vi "UHR-Fleezers Control (host) - 10.8MV_trial1.vi"() -> ()   [LabVIEW 2010] (continued)
        n694 = xnode "Read/Write Control"("FPGA VI Reference In"=w3318, "error in"=w3316, "Green interlace ON count"="GI Frequency, ON count", "Green interlace OFF count"="GI Frequency, OFF count", "Green interlace ON count 2"="GI Frequency, ON count", "Green interlace OFF count 2"="GI Frequency, OFF count", "Green FB Count"="Green FB Count") -> ("error out"=w3317:errorcluster)  [unwired: 1 out]
      }
      event "Number of F/B Scans (AOD)", "Scan Speed (nm/s)", "Scan BD", "Initial delta (MHz)", "Step Size (nm)", "Scan Range (nm)": Value Change {
        w3497 = 123.0  # AOM cal (nm/MHz)
        n695 = event-data() -> ()  [unwired: 7 out]
        n696 = local read "BD 1 Frequency 1 (MHz)"() -> (w3480:dbl)
        n697 = local read "AOM X Cal (nm/MHz)"() -> (w3472:dbl)
        n698 = local read "X RF Frequency Limits (MHz)"() -> (w3484:T16)
        n699 = local read "Y RF Frequency Limits (MHz)"() -> (w3481:T16)
        n700 = local read "BD 2 Frequency 1 (MHz)"() -> (w3486:dbl)
        n701 = Negate(x="Scan Range (nm)") -> (-x=w3450:dbl)
        n702 = Divide(x=w3450, y=w3472) -> (x/y=w3454:dbl)
        n703 = Select(t=w3484, s="Scan BD", f=w3481) -> (s? t:f=w3483:T16)
        n704 = Select(t=w3480, s="Scan BD", f=w3486) -> (s? t:f=w3485:dbl)
        n705 = Unbundle By Name(w3483) -> ("Maximum"=w3492:dbl, "Minimum"=w3491:dbl)
        n706 = Add(x=w3454, y=w3485) -> (x+y=w3489:dbl)
        n707 = Divide(x=w3450, y="Step Size (nm)") -> (x/y=w3469:dbl)
        n708 = Divide(x="Step Size (nm)", y=w3472) -> (x/y=w3478:dbl)
        n709 = Absolute Value(x=w3469) -> (abs(x)=w3453:dbl)
        n710 = Sign(1:w3450) -> (0:w3451:dbl)
        n711 = In Range and Coerce(upper limit=w3492, x=w3489, lower limit=w3491) -> (coerced(x)=w3488:dbl, In Range?=w3490:bool)
        n712 = To Unsigned Quad Integer(1:w3453) -> (0:w3468:u64)
        "Scan steps (AOD)" <- w3468
        n713 = call "IR AOM freq to word.vi"("Frequency In (MHz)"=w3478) -> ("Frequency Word Out (double)"=w3475:dbl)
        n714 = Multiply(x=w3451, y=w3475) -> (x*y=w3452:dbl)
        n715 = Subtract(x=w3489, y=w3488) -> (x-y=w3487:dbl)
        n716 = To Quad Integer(1:w3452) -> (0:w3474:i64)
        "Incr. int (AOD)" <- w3474
        n717 = Subtract(x=w3454, y=w3487) -> (x-y=w3473:dbl)
        "Scan Range (MHz)" <- w3473
        n718 = Select(t=w3454, s=w3490, f=w3473) -> (s? t:f=w3493:dbl)
        n719 = Multiply(x=w3473, y=w3472) -> (x*y=w3471:dbl)
        n720 = Decrement(x=w3468) -> (x-1=w3521:u64)
        n721 = Negate(x=w3471) -> (-x=w3467:dbl)
        n722 = local write "Scan Range (nm)"(w3467) -> ()
        n723 = Divide(x=w3493, y=w3521) -> (x/y=w3477:dbl)
        "Scan Increment (MHz)" <- w3477
        n724 = call "IR AOM freq to word.vi"("Frequency In (MHz)"=w3477) -> ("Frequency Word Out (double)"=w3476:dbl)
        n725 = Divide(x="Step Size (nm)", y="Scan Speed (nm/s)") -> (x/y=w3464:dbl)
        n726 = To Quad Integer(1:w3476) -> ()  [unwired: 1 out]
        n727 = local read "Number Interlace Sets"() -> (w3448:u8)
        n728 = local read "AI Count (ticks)"() -> (w3449:u32)
        n729 = local read "Total Counts (ticks)"() -> (w3447:u32)
        n730 = local read "# Samples/trap"() -> (w3479:u32)
        n731 = Multiply(x=w3449, y=w3448) -> (x*y=w3446:u32)
        n732 = Divide(x=w3447, y=w3446) -> (x/y=w3445:dbl)
        n733 = Select(t=w3480, s="Scan BD", f=w3486) -> (s? t:f=w3518:dbl)
        "Initial freq. (MHz)" <- w3518
        n734 = Add(x=w3493, y=w3518) -> (x+y=→"Final freq. (MHz)":dbl)
        n735 = Divide(x=w3447, y=40000000.0) -> (x/y=w3463:dbl)
        n736 = Divide(x=w3464, y=w3463) -> (x/y=w3462:dbl)
        n737 = To Unsigned Quad Integer(1:w3462) -> (0:w3437:u64)
        n738 = Quotient & Remainder(x=w3437, y=u64 2) -> (x-y*floor(x/y)=w3441:u64)  [unwired: 1 out]
        n739 = Equal?(x=w3441, y=u64 0) -> (x = y?=w3439:bool)
        n740 = Decrement(x=w3437) -> (x-1=w3438:u64)
        n741 = Select(t=w3437, s=w3439, f=w3438) -> (s? t:f=w3436:u64)
        "Cycles/step (AOD)" <- w3436
        n742 = xnode "Read/Write Control"("FPGA VI Reference In"=w3529, "error in"=w3528, "Scan steps"=w3468, "Number of scans"="Number of F/B Scans (AOD)", "Cycles per step"=w3436, "Scan freq.  increment"=w3474, "Scan BD"="Scan BD") -> ("error out"=w3527:errorcluster)  [unwired: 1 out]
        n743 = Multiply(x=w3468, y=w3436) -> (x*y=w3522:u64)
        n744 = Multiply(x=w3522, y=u64 2) -> (x*y=w3444:u64)
        n745 = Multiply(x=w3445, y=w3444) -> (x*y=w3443:dbl)
        "Data points/scan (f/b)" <- w3443
        n746 = Multiply(x=w3443, y="Number of F/B Scans (AOD)") -> (x*y=w3525:dbl)
        "Data points/scans" <- w3525
        n747 = Divide(x=w3525, y=w3479) -> (x/y=→"N sets should be saved":dbl)
        n748 = Multiply(x=w3522, y=w3463) -> (x*y=w3461:dbl)
        "Time/Scan (s) (AOD)" <- w3461
        n749 = Select(t=w3493, s="Scan BD", f=0.0) -> (s? t:f=w3519:dbl)
        n750 = Select(t=0.0, s="Scan BD", f=w3493) -> (s? t:f=w3515:dbl)
        n751 = local read "BD 2 Frequency 2 (MHz)"() -> (w3511:dbl)
        n752 = local read "BD 1 Frequency 2 (MHz)"() -> (w3514:dbl)
        n753 = Add(x=w3515, y=w3486) -> (x+y=w3512:dbl)
        n754 = Add(x=w3480, y=w3519) -> (x+y=w3513:dbl)
        n755 = Multiply(x=w3461, y=2.0) -> (x*y=w3460:dbl)
        n756 = Multiply(x=w3460, y="Number of F/B Scans (AOD)") -> (x*y=w3457:dbl)
        n757 = Divide(x=w3457, y=60.0) -> (x/y=→"Time to Finish All (min)":dbl)
        n758 = Add(x="Trap 2 Bead Size (nm)", y="Trap 1 Bead Size (nm)") -> (x+y=w3501:dbl)
        n759 = local read "Initial delta (MHz)"() -> (w3498:dbl)
        n760 = Divide(x=w3501, y=2.0) -> (x/y=w3495:dbl)
        n761 = Subtract(x=w3512, y=w3511) -> (x-y=w3509:dbl)
        n762 = Subtract(x=w3513, y=w3514) -> (x-y=w3510:dbl)
        n763 = Square(x=w3509) -> (x^2=w3508:dbl)
        n764 = Square(x=w3510) -> (x^2=w3507:dbl)
        n765 = Add(x=w3507, y=w3508) -> (x+y=w3506:dbl)
        n766 = Square Root(x=w3506) -> (sqrt(x)=w3505:dbl)
        "Final delta (MHz)" <- w3505
        n767 = Multiply(x=w3497, y=w3505) -> (x*y=w3504:dbl)
        n768 = Multiply(x=w3498, y=w3497) -> (x*y=w3496:dbl)
        n769 = Subtract(x=w3496, y=w3495) -> (x-y=→"Initial sep (nm)":dbl)
        n770 = Subtract(x=w3504, y=w3495) -> (x-y=→"Final sep (nm)":dbl)
      }
      event "Raster Scanning...": Value Change {
        n771 = event-data() -> ("NewVal"=w3666:bool)  [unwired: 6 out]
        n772 = case shown="True" w3666 {
          frame False {
          }
          frame True {
            n773 = property on="BD 1 Frequency 1 (MHz)" class="DigNum (strict)"("Val(Sgnl)"=65.0 ("Value (Signaling)")) -> ()  [unwired: 2 in, 2 out]
          }
        }
      }
      event "Freq or Amp switch first", "Swap F1 and F2", "Freq switch delay", "Amp switch delay": Value Change {
        n774 = event-data() -> ()  [unwired: 7 out]
        n775 = local read "Freq or Amp switch first"() -> (w3668:bool)
        n776 = local read "Amp switch delay"() -> (w3669:u16)
        n777 = local read "Freq switch delay"() -> (w3671:u16)
        n778 = local read "Swap F1 and F2"() -> (w3670:bool)
        n779 = xnode "Read/Write Control"("FPGA VI Reference In"=w3674, "error in"=w3673, "Freq switch delay"=w3671, "Swap F1 and F2"=w3670, "Amp switch delay"=w3669, "Freq or Amp switch first"=w3668) -> ("error out"=w3672:errorcluster)  [unwired: 1 out]
      }
      event "Scan steps (MCL)", "Number of scans (MCL)", "Scan Range (V)\n(of steps)", "2D or 1D Scan", "N APD Samp/step", "Fast Scan Dir", "Continuous MCL Scanning", "Scan lines (y)": Value Change {
        w3775 = 32767.0 ("y")
        n780 = event-data() -> ()  [unwired: 7 out]
        n781 = Select(t="Scan lines (y)", s="2D or 1D Scan", f="Number of scans (MCL)") -> (s? t:f=w3780:u64)
        n782 = Decrement(x="Scan steps (MCL)") -> (x-1=w3796:u64)
        n783 = Divide(x="Scan Range (V)\n(of steps)", y=w3796) -> (x/y=w3795:dbl)
        "Desired Scan Incr (V)" <- w3795
        n784 = local read "APD Integration Time (s)"() -> (w3788:dbl)
        n785 = Multiply(x=w3795, y=w3775) -> (x*y=w3804:dbl)
        n786 = Divide(x=w3804, y=10.0) -> (x/y=w3794:dbl)
        "Desired incr (int)" <- w3794
        n787 = local read "Update Count (MCL)"() -> (w3800:u32)
        n788 = Round Toward -Infinity(1:w3794) -> (0:w3803:dbl)
        n789 = To Word Integer(number=w3803) -> (16bit integer=w3778:i16)
        "Actual Incr. int (MCL)" <- w3778
        n790 = Multiply(x=w3788, y=40000000.0) -> (x*y=w3801:dbl)
        n791 = Divide(x=w3801, y=w3800) -> (x/y=w3799:dbl)
        n792 = Multiply(x=i16 10, y=w3778) -> (x*y=w3776:i16)
        n793 = Multiply(x="N APD Samp/step", y=w3799) -> (x*y=w3798:dbl)
        "Cycles/step (MCL)" <- w3798
        n794 = Divide(x=w3776, y=w3775) -> (x/y=→"Actual MCL Inc (V)":dbl)
        n795 = Multiply(x="N APD Samp/step", y="Scan steps (MCL)") -> (x*y=w3790:dbl)
        n796 = local read "APD Samples/FIFO Acq."() -> (w3787:dbl)
        n797 = Multiply(x=w3790, y=u64 2) -> (x*y=w3789:dbl)
        "Data points/scan (f+b)" <- w3789
        n798 = Multiply(x=w3789, y=w3780) -> (x*y=w3807:dbl)
        "Data points/scans (MCL)" <- w3807
        n799 = Multiply(x=w3788, y=w3789) -> (x*y=w3781:dbl)
        "Time/f+b scan (s) (MCL)" <- w3781
        n800 = Divide(x=w3807, y=w3787) -> (x/y=→"N sets should be saved (MCL)":dbl)
        n801 = Multiply(x=w3781, y=w3780) -> (x*y=→"Total Time (s)":dbl)
        n802 = Not(x="Fast Scan Dir") -> (.not. x?=w3785:bool)
        n803 = xnode "Read/Write Control"("FPGA VI Reference In"=w3811, "error in"=w3810, "Scan steps (MCL)"="Scan steps (MCL)", "Number of scans (MCL)"=w3780, "Cycles per step (MCL)"=w3798, "Scan freq.  increment (MCL)"=w3778, "1D or 2D Scan?"="2D or 1D Scan", "MCL Scan Axis"=w3785, "Cont. Scan (MCL)"="Continuous MCL Scanning") -> ("error out"=w3809:errorcluster)  [unwired: 1 out]
      }
      event "Read Cal": Value Change {
        w3985 = 1000.0 ("y")
        n804 = event-data() -> ()  [unwired: 7 out]
        n805 = local read "Save file name"() -> (w4010:path)
        n806 = local write "Read Cal"(FALSE ("Read Cal")) -> ()
        n807 = Strip Path(path=w4010) -> (stripped path=w4009:path)  [unwired: 1 out]
        n808 = Path To String(path=w4009) -> (string=w4008:string)
        n809 = Concatenate Strings(w4008, "\\current.cal" ("string")) -> (w4006:string)
        n810 = String To Path(string=w4006) -> (path=w4005:path)
        n811 = Open/Create/Replace File(file path (use dialog)=w4005, operation (0:open)=T25."open", access (0:read/write)=enum16{"read/write", "read-only", "write-only"}."read-only") -> (refnum out=w4013:refnum<file>, error out=w3999:errorcluster)  [unwired: 1 in, 3 out]
        n812 = Deny Access(4:w3999, 7:w4013) -> (0:w3998:errorcluster, 3:w4004:refnum<file>)  [unwired: 1 out]
        n813 = Read from Binary File(5:0.0, 8:w3998, 9:T31."big-endian, network order" ("byte order (0:big-endian, network order)"), 10:-1 ("count (1)"), 11:w4004) -> (0:w3997:errorcluster, 2:w3995:dbl[], 3:w4000:refnum<file>)  [unwired: 2 out]
        n814 = Array To Cluster(array=w3995) -> (cluster=w3994:T33)
        n815 = Unbundle(w3994) -> ("[0]"=w3993:dbl, "[1]"=w3992:dbl, "[2]"=w3991:dbl, "[3]"=w3990:dbl, "[4]"=w3989:dbl, "[5]"=w3988:dbl)
        n816 = Close File(refnum=w4000, error in=w3997) -> (error out=→"Read cal error":errorcluster)  [unwired: 1 out]
        n817 = Multiply(x=w3988, y=w3985) -> (x*y=w3986:dbl)
        n818 = local write "T2 kappa_x (pN/nm)"(w3990) -> ()
        n819 = local write "T1 kappa_x (pN/nm)"(w3991) -> ()
        n820 = local write "T1 alpha_x (nm/V)"(w3993) -> ()
        n821 = local write "T2 alpha_x (nm/V)"(w3992) -> ()
        n822 = Multiply(x=w3989, y=w3985) -> (x*y=w3987:dbl)
        n823 = local write "T1 offset_x (mV)"(w3987) -> ()
        n824 = local write "T2 offset_x (mV)"(w3986) -> ()
      }
      event "Abort MCL Scan": Value Change {
        n825 = event-data() -> ()  [unwired: 7 out]
        n826 = local write "MCL Scanning"(FALSE ("MCL Scanning")) -> ()
        n827 = xnode "Read/Write Control"("FPGA VI Reference In"=w4018, "error in"=w4017, "Abort scan (MCL)"="Abort MCL Scan") -> ("error out"=w4016:errorcluster)  [unwired: 1 out]
      }
      event "Update Count (MCL)": Value Change {
        n828 = event-data() -> ()  [unwired: 7 out]
        n829 = xnode "Read/Write Control"("FPGA VI Reference In"=w4060, "error in"=w4059, "MCL count"="Update Count (MCL)") -> ("error out"=w4058:errorcluster)  [unwired: 1 out]
      }
      event "Phase adjust (MCL)", "+ phase (MCL)", "- phase (MCL)": Value Change {
        n830 = event-data() -> ()  [unwired: 7 out]
        n831 = Negate(x="Phase adjust (MCL)") -> (-x=w4106:i16)
        n832 = Select(t=w4106, s="- phase (MCL)", f="Phase adjust (MCL)") -> (s? t:f=w4104:i16)
        n833 = Or(x="- phase (MCL)", y="+ phase (MCL)") -> (x .or. y?=w4099:bool)
        n834 = xnode "Read/Write Control"("FPGA VI Reference In"=w4108, "error in"=w4107, "Phase count adjustment (MCL)"=w4104) -> ("FPGA VI Reference Out"=w4100:T19, "error out"=w4101:errorcluster)
        n835 = xnode "Read/Write Control"("FPGA VI Reference In"=w4100, "error in"=w4101, "+ phase (MCL)"=w4099) -> ("error out"=w4098:errorcluster)  [unwired: 1 out]
      }
      event "Abort AOD Scan": Value Change {
        n836 = event-data() -> ()  [unwired: 7 out]
        n837 = xnode "Read/Write Control"("FPGA VI Reference In"=w4187, "error in"=w4186, "Abort scan"="Abort AOD Scan") -> ("error out"=w4185:errorcluster)  [unwired: 1 out]
      }
      event "Continuous AOD Scanning": Value Change {
        n838 = event-data() -> ()  [unwired: 7 out]
        n839 = xnode "Read/Write Control"("FPGA VI Reference In"=w4229, "error in"=w4228, "Cont. Scan"="Continuous AOD Scanning") -> ("error out"=w4227:errorcluster)  [unwired: 1 out]
      }
      event "Index": Value Change {
        n840 = event-data() -> ()  [unwired: 7 out]
        n841 = call "Create new save file.vi"("Insert"="", "Ext"=".dat" ("string"), "Index In"="Index") -> ("Path Out"=→"Save file name":path, "Index Out"=w4268:dbl)
        "Save index" <- w4268
        n842 = local write "Index"(w4268) -> ()
      }
      event "AO1", "AO2": Value Change {
        w4283 = 10.0 ("y")
        w4282 = 32767.0 ("y")
        n843 = event-data() -> ()  [unwired: 7 out]
        n844 = local read "AO2"() -> (w4281:dbl)
        n845 = local read "AO1"() -> (w4278:dbl)
        n846 = Multiply(x=w4278, y=w4282) -> (x*y=w4277:dbl)
        n847 = Multiply(x=w4281, y=w4282) -> (x*y=w4280:dbl)
        n848 = Divide(x=w4277, y=w4283) -> (x/y=w4276:dbl)
        n849 = Divide(x=w4280, y=w4283) -> (x/y=w4279:dbl)
        n850 = To Word Integer(number=w4276) -> (16bit integer=w4284:i16)
        n851 = To Word Integer(number=w4279) -> (16bit integer=w4285:i16)
        n852 = xnode "Read/Write Control"("FPGA VI Reference In"=w4275, "error in"=w4274, "AO1"=w4284, "AO2"=w4285) -> ("error out"=w4273:errorcluster)  [unwired: 1 out]
      }
      event "Inject Bottom": Value Change {
        n853 = event-data() -> ()  [unwired: 7 out]
        n854 = disable-structure shown="Enabled" {
          disable-tunnel: "Inject Bottom" -> [w4344 w4384]
          frame Disabled {
            n855 = local read "Chemyx Syringe Pump Serial Port"() -> (w4345:refnum<visa-resource-name>)
            n856 = local read "Pump write delay (ms)"() -> (w4346:dbl)
            n857 = case shown="True" w4344 {
              tunnel: w4346 -> [w4352 w4366]
              tunnel: w4345 -> [w4349 w4365]
              frame False {
                n858 = flat-sequence {
                  tunnel: w4349 -> [w4353]
                  tunnel: [w4353] -> w4350
                  tunnel: w4352 -> [_]
                  tunnel: [w4356] -> w4351
                  tunnel: w4350 -> [w4356]
                  tunnel: w4351 -> [w4357]
                  tunnel: [w4357] -> w4347
                  tunnel: [w4359] -> w4348
                  tunnel: w4347 -> [w4359]
                  tunnel: w4348 -> [w4361]
                  frame #0 {
                    n859 = call "Write to pump.vi"("string"="enter pump1", "VISA resource name"=w4353) -> ()  [unwired: 1 out]
                  }
                  frame #1 {
                    n860 = Wait (ms)(milliseconds to wait="Pump pause delay (ms)") -> ()  [unwired: 1 out]
                  }
                  frame #2 {
                    n861 = call "Write to pump.vi"("string"="stop", "VISA resource name"=w4357) -> ()  [unwired: 1 out]
                  }
                  frame #3 {
                    n862 = Wait (ms)(milliseconds to wait=u32 500) -> ()  [unwired: 1 out]
                  }
                  frame #4 {
                    n863 = call "Write to pump.vi"("string"="stop", "VISA resource name"=w4361) -> ()  [unwired: 1 out]
                  }
                }
              }
              frame True {
                n864 = flat-sequence {
                  tunnel: w4365 -> [w4375]
                  tunnel: w4366 -> [w4370]
                  tunnel: w4366 -> [w4377]
                  tunnel: w4365 -> [w4378]
                  tunnel: [w4378] -> w4363
                  tunnel: [w4380] -> w4364
                  tunnel: w4363 -> [w4380]
                  tunnel: w4364 -> [w4382]
                  frame #0 {
                    n865 = local read "All Pump Parameters"() -> (w4369:T5)
                    n866 = Unbundle By Name(w4369) -> ("Pump 1"=w4376:T34)
                    n867 = call "Set pump parameters.vi"("Pump write delay (ms)"=w4370, "Volume (uL)"="Ch 2 Inject Volume (uL)", "Rate (uL/h)"="Ch 1 Inject Rate (ul/h)", "Units"=4.0, "Pump #"=1.0, "Pump Parameters In"=w4376, "VISA resource name"=w4375) -> ("Pump Parameters Out"=w4368:T34)  [unwired: 3 in]
                    n868 = Bundle By Name(cluster=w4369, "Pump 1"=w4368) -> (w4367:T5)
                    n869 = local write "All Pump Parameters"(w4367) -> ()
                  }
                  frame #1 {
                    n870 = Wait (ms)(milliseconds to wait=w4377) -> ()  [unwired: 1 out]
                  }
                  frame #2 {
                    n871 = call "Write to pump.vi"("string"="start", "VISA resource name"=w4378) -> ()  [unwired: 1 out]
                  }
                  frame #3 {
                    n872 = Wait (ms)(milliseconds to wait=u32 500) -> ()  [unwired: 1 out]
                  }
                  frame #4 {
                    n873 = call "Write to pump.vi"("string"="start", "VISA resource name"=w4382) -> ()  [unwired: 1 out]
                  }
                }
              }
            }
          }
          frame Enabled {
            n874 = call "hamilton_controller.vi"("Open?"=w4384, "valve"=enum16{"A", "B", "C", "D", "ALL"}."B", "action"=T22."MOVE VALVE") -> ()  [unwired: 8 in, 1 out]
          }
        }
      }
      event "Inject Top": Value Change {
        n875 = event-data() -> ()  [unwired: 7 out]
        n876 = disable-structure shown="Disabled" {
          disable-tunnel: "Inject Top" -> [_ w4428]
          frame Disabled {
            n877 = local read "Pump write delay (ms)"() -> (w4389:dbl)
            n878 = case shown="False" w4390 {
              tunnel: w4389 -> [w4396 w4410]
              tunnel: "Chemyx Syringe Pump Serial Port" -> [w4393 w4409]
              frame False {
                n879 = flat-sequence {
                  tunnel: w4393 -> [w4397]
                  tunnel: [w4397] -> w4394
                  tunnel: w4396 -> [_]
                  tunnel: [w4400] -> w4395
                  tunnel: w4394 -> [w4400]
                  tunnel: w4395 -> [w4401]
                  tunnel: [w4401] -> w4391
                  tunnel: [w4403] -> w4392
                  tunnel: w4391 -> [w4403]
                  tunnel: w4392 -> [w4405]
                  frame #0 {
                    n880 = call "Write to pump.vi"("string"="enter pump3", "VISA resource name"=w4397) -> ()  [unwired: 1 out]
                  }
                  frame #1 {
                    n881 = local read "Pump pause delay (ms)"() -> (w4399:u32)
                    n882 = Wait (ms)(milliseconds to wait=w4399) -> ()  [unwired: 1 out]
                  }
                  frame #2 {
                    n883 = call "Write to pump.vi"("string"="stop", "VISA resource name"=w4401) -> ()  [unwired: 1 out]
                  }
                  frame #3 {
                    n884 = Wait (ms)(milliseconds to wait=u32 0) -> ()  [unwired: 1 out]
                  }
                  frame #4 {
                    n885 = call "Write to pump.vi"("string"="stop", "VISA resource name"=w4405) -> ()  [unwired: 1 out]
                  }
                }
              }
              frame True {
                n886 = flat-sequence {
                  tunnel: w4409 -> [w4419]
                  tunnel: w4410 -> [w4414]
                  tunnel: w4410 -> [w4421]
                  tunnel: w4409 -> [w4422]
                  tunnel: [w4422] -> w4407
                  tunnel: [w4425] -> w4408
                  tunnel: w4407 -> [w4425]
                  tunnel: w4408 -> [w4426]
                  frame #0 {
                    n887 = local read "All Pump Parameters"() -> (w4413:T5)
                    n888 = Unbundle By Name(w4413) -> ("Pump 3"=w4420:T34)
                    n889 = call "Set pump parameters.vi"("Pump write delay (ms)"=w4414, "Volume (uL)"="Ch 3 Inject Volume (uL)", "Rate (uL/h)"="Ch 3 Inject Rate (ul/h)", "Units"=4.0, "Pump #"=3.0, "Pump Parameters In"=w4420, "VISA resource name"=w4419) -> ("Pump Parameters Out"=w4412:T34)  [unwired: 3 in]
                    n890 = Bundle By Name(cluster=w4413, "Pump 3"=w4412) -> (w4411:T5)
                    n891 = local write "All Pump Parameters"(w4411) -> ()
                  }
                  frame #1 {
                    n892 = Wait (ms)(milliseconds to wait=w4421) -> ()  [unwired: 1 out]
                  }
                  frame #2 {
                    n893 = call "Write to pump.vi"("string"="start", "VISA resource name"=w4422) -> ()  [unwired: 1 out]
                  }
                  frame #3 {
                    n894 = Wait (ms)(milliseconds to wait=u32 500) -> ()  [unwired: 1 out]
                  }
                  frame #4 {
                    n895 = call "Write to pump.vi"("string"="start", "VISA resource name"=w4426) -> ()  [unwired: 1 out]
                  }
                }
              }
            }
          }
          frame Enabled {
            n896 = call "hamilton_controller.vi"("Open?"=w4428, "valve"=enum16{"A", "B", "C", "D", "ALL"}."A", "action"=T22."MOVE VALVE") -> ()  [unwired: 8 in, 1 out]
          }
        }
      }
      event "Inject Valve B": Value Change {
        n897 = event-data() -> ()  [unwired: 7 out]
        n898 = disable-structure shown="Enabled" {
          disable-tunnel: "Inject Valve B" -> [w4432 w4452]
          frame Disabled {
            n899 = local read "Pump write delay (ms)"() -> (w4434:dbl)
            n900 = flat-sequence {
              tunnel: w4433 -> [w4447]
              tunnel: w4434 -> [w4443]
              tunnel: w4432 -> [_]
              tunnel: w4434 -> [w4449]
              tunnel: w4433 -> [w4450]
              frame #0 {
                n901 = local read "All Pump Parameters"() -> (w4442:T5)
                n902 = Multiply(x=60.0, y="Flush Center Ch Rate (ul/m)") -> (x*y=w4439:dbl)
                n903 = Unbundle By Name(w4442) -> ("Pump 2"=w4448:T34)
                n904 = call "Set pump parameters.vi"("Pump write delay (ms)"=w4443, "Volume (uL)"="Flush Center Ch Volume (uL)", "Rate (uL/h)"=w4439, "Units"=3.0, "Pump #"=2.0, "Pump Parameters In"=w4448, "VISA resource name"=w4447) -> ("Pump Parameters Out"=w4441:T34)  [unwired: 3 in]
                n905 = Bundle By Name(cluster=w4442, "Pump 2"=w4441) -> (w4440:T5)
                n906 = local write "All Pump Parameters"(w4440) -> ()
                n907 = Add(x="Flush Center Ch Volume (uL)", y="Total Volume\nFlushed (uL)") -> (x+y=w4436:dbl)
                n908 = local write "Total Volume\nFlushed (uL)"(w4436) -> ()
              }
              frame #1 {
                n909 = Wait (ms)(milliseconds to wait=w4449) -> ()  [unwired: 1 out]
              }
              frame #2 {
                n910 = call "Write to pump.vi"("string"="start", "VISA resource name"=w4450) -> ()  [unwired: 1 out]
              }
            }
            n911 = local read "Chemyx Syringe Pump Serial Port"() -> (w4433:refnum<visa-resource-name>)
          }
          frame Enabled {
            n912 = call "hamilton_controller.vi"("Open?"=w4452, "valve"=enum16{"A", "B", "C", "D", "ALL"}."B", "action"=T22."MOVE VALVE") -> ()  [unwired: 8 in, 1 out]
          }
        }
      }
      event "Sample Channel Flow": Value Change {
        n913 = event-data() -> ()  [unwired: 7 out]
        n914 = call "hamilton_controller.vi"("Open?"="Sample Channel Flow", "valve"=enum16{"A", "B", "C", "D", "ALL"}."C", "action"=T22."MOVE VALVE") -> ()  [unwired: 8 in, 1 out]
      }
      event "Flip Green Filter": Value Change {
        n915 = event-data() -> ()  [unwired: 7 out]
        n916 = Not(x="Flip Green Filter") -> (.not. x?=w4458:bool)
        n917 = local write "Flip Green Filter"(w4458) -> ()
        n918 = flat-sequence {
          tunnel: w4466 -> [w4471]
          tunnel: w4465 -> [w4470]
          tunnel: [w4468] -> w4463
          tunnel: [w4467] -> w4462
          tunnel: [w4511] -> w4461
          tunnel: w4463 -> [w4511]
          tunnel: [w4510] -> w4460
          tunnel: w4462 -> [w4510]
          tunnel: w4461 -> [w4515]
          tunnel: w4460 -> [w4514]
          tunnel: [w4513] -> w4464
          frame #0 {
            n919 = xnode "Read/Write Control"("FPGA VI Reference In"=w4471, "error in"=w4470, "Green Filter Flipper"=TRUE) -> ("FPGA VI Reference Out"=w4468:T19, "error out"=w4467:errorcluster)
          }
          frame #1 {
            n920 = Wait (ms)(milliseconds to wait=u32 100) -> ()  [unwired: 1 out]
          }
          frame #2 {
            n921 = xnode "Read/Write Control"("FPGA VI Reference In"=w4515, "error in"=w4514, "Green Filter Flipper"=FALSE) -> ("error out"=w4513:errorcluster)  [unwired: 1 out]
          }
        }
      }
      event "Pump 1 contents", "Pump 3 contents": Value Change {
        n922 = event-data() -> ()  [unwired: 7 out]
        n923 = local read "Pump 1 contents"() -> (→"Pump 1 cont disp":string)
        n924 = local read "Pump 3 contents"() -> (→"Pump 3 cont disp":string)
      }
      event "Reset Trap Pos. FB": Value Change {
        n925 = event-data() -> ()  [unwired: 7 out]
        n926 = xnode "Read/Write Control"("FPGA VI Reference In"=w4559, "error in"=w4558, "Trap Pos. FB Reset"="Reset Trap Pos. FB") -> ()  [unwired: 2 out]
      }
      event "Trap Pos. FB ON": Value Change {
        n927 = event-data() -> ()  [unwired: 7 out]
        n928 = xnode "Read/Write Control"("FPGA VI Reference In"=w4600, "error in"=w4599, "Force feedback"="Trap Pos. FB ON") -> ()  [unwired: 2 out]
      }
      event "Trap Pos. FB Range", "Trap Pos. FB Gains", "Trap Pos. FB Mult Factor", "Trap Pos. FB Offset Factor", "Trap Pos FB Negate Action", "Trap Pos FB Monitor\nT1 or T2": Value Change {
        n929 = event-data() -> ()  [unwired: 7 out]
        n930 = xnode "Read/Write Control"("FPGA VI Reference In"=w4647, "error in"=w4646, "Trap Pos. FB Range"="Trap Pos. FB Range", "Trap Pos. FB Gains"="Trap Pos. FB Gains", "Trap Pos. FB Mult Factor"="Trap Pos. FB Mult Factor", "Trap Pos. FB Offset Factor"="Trap Pos. FB Offset Factor", "Trap Pos FB Negate Action"="Trap Pos FB Negate Action", "Trap Pos FB Monitor T1 or T2"="Trap Pos FB Monitor\nT1 or T2", "AI1 X Scale"="Trap Pos. AI1 X Pre-scale") -> ()  [unwired: 2 out]
      }
      event "Trap Pos FB SP": Value Change {
        n931 = event-data() -> ()  [unwired: 7 out]
        n932 = xnode "Read/Write Control"("FPGA VI Reference In"=w4835, "error in"=w4834, "Trap Pos. FB SP"="Trap Pos FB SP") -> ()  [unwired: 2 out]
      }
      event "Set SP to Reading": Value Change {
        n933 = event-data() -> ()  [unwired: 7 out]
        n934 = local read "Trap Pos FB Monitor\nT1 or T2"() -> (w4888:bool)
        n935 = local read "Trap X AI1 (DMA)"() -> (w4891:T13)
        n936 = local read "Trap X (AI1)"() -> (w4894:T10)
        n937 = Unbundle By Name(w4894) -> ("Trap 1"=w4893:fxp<+/-,16,1>, "Trap 2"=w4892:fxp<+/-,16,1>)
        n938 = Unbundle By Name(w4891) -> ("Set 1"=w4890:fxp<+/-,16,1>, "Set 2"=w4889:fxp<+/-,16,1>)
        n939 = Select(t=w4893, s=w4888, f=w4892) -> (s? t:f=w4887:fxp<+/-,16,1>)
        n940 = Select(t=w4890, s=w4888, f=w4889) -> (s? t:f=w4886:fxp<+/-,16,1>)
        n941 = Not(x="Set SP Using...") -> (.not. x?=w4881:bool)
        n942 = Select(t=w4887, s=w4881, f=w4886) -> (s? t:f=w4882:fxp<+/-,16,1>)
        n943 = xnode "Read/Write Control"("FPGA VI Reference In"=w4884, "error in"=w4883, "Trap Pos. FB SP"=w4882) -> ()  [unwired: 2 out]
        n944 = local write "Trap Pos FB SP"(w4882) -> ()
      }
      event "Trap Pos. FB Out Scale 2^n": Value Change {
        n945 = event-data() -> ()  [unwired: 7 out]
        n946 = Scale By Power Of 2(n="Trap Pos. FB Out Scale 2^n", x=ext 1.0) -> (x*2^n=w4941:ext)
        n947 = property on="Trap Pos. FB Mult Factor" class="DigNum (strict)"("Val(Sgnl)"=w4941) -> ()  [unwired: 2 in, 2 out]
      }
      event "Trap Pos FB Int Count": Value Change {
        n948 = event-data() -> ()  [unwired: 7 out]
        n949 = xnode "Read/Write Control"("FPGA VI Reference In"=w4946, "error in"=w4945, "Trap Pos FB Int Count"="Trap Pos FB Int Count") -> ()  [unwired: 2 out]
      }
    }
    "error out 2" <- w1271
    n950 = node-c288() -> ()  [unwired: 1 in, 1 out]
  }
  n951 = timed-loop "Run Scripts, including: stage motion" {
    timing: w69 -> [_]
    timing-out: [_] -> w68
    tunnel: w24 -> [_]
    stop <- w4985 stop-if-true
    n952 = node-c288() -> ()  [unwired: 1 in, 1 out]
    n953 = event shown="[2] \"Cal/Data Acq. Spot\": Value Change" {
      selector: _ -> [_ _ _ _ _ _ _ _ _ _ _ _]
      dyn-events: _ -> [_ _ _ _ _ _ _ _ _ _ _ _]
      timeout: 50 -> [_ _ _ _ _ _ _ _ _ _ _ _]
      tunnel: ["Move Cap. 1 (DNA Top)" _ "Cal/Data Acq. Spot" "Dump Beads" "Dip for Protein" _ "Got ADig bead" "Got DNA bead" "Take Stepping Data" _ "Take Detection Laser\nImage" _] -> _
      tunnel: [_ _ _ _ _ _ _ _ _ _ _ w5189] -> w4985
      event "Move Cap. 1 (DNA Top)": Value Change {
        n954 = event-data() -> ()  [unwired: 1 in, 5 out]
        n955 = local write "Move Cap. 1 (DNA Top)"(FALSE ("Move Cap. 1 (DNA Right)")) -> ()
        n956 = flat-sequence {
          tunnel: "Cap 1 Samp Flow ON" -> [w4991]
          frame #0 {
            n957 = local write "Stage Moving"(FALSE ("Stage Moving")) -> ()
            n958 = case "stop flow" shown="True" w4991 {
              frame False {
              }
              frame True {
                n959 = call "hamilton_controller.vi"("Open?"=FALSE, "valve"=enum16{"A", "B", "C", "D", "ALL"}."C", "action"=T22."MOVE VALVE") -> ()  [unwired: 8 in, 1 out]
              }
            }
            n960 = case shown="True" TRUE {
              tunnel: "Cap 1 T ON" -> [w5000 w5001]
              frame False {
                n961 = property on="Trap 1 (ON/OFF)" class="Bool (strict)"("Val(Sgnl)"=w5000) -> ()  [unwired: 2 in, 2 out]
              }
              frame True {
                n962 = property on="Trap 2 (ON/OFF)" class="Bool (strict)"("Val(Sgnl)"=w5001) -> ()  [unwired: 2 in, 2 out]
              }
            }
            n963 = call <vilib>:"Beep.vi"() -> ()  [unwired: 3 in, 9 out]
            n964 = case shown="True" "Cap 1 Flow ON" {
              frame False {
              }
              frame True {
                n965 = property on="Inject Top" class="Bool (strict)"("Val(Sgnl)"=TRUE ("Value (Signaling)")) -> ()  [unwired: 2 in, 2 out]
              }
            }
          }
        }
      }
      event Timeout {
        n966 = event-data() -> ()  [unwired: 1 in, 2 out]
      }
      event "Cal/Data Acq. Spot": Value Change {
        # "wait for calibration file\nto be written"
        # "signal save cal true\nthis tells the data \nacquisition loop to\nstart sending the data\nto a calibration file"
        # "separate traps to\nthe desired trap delta"
        # "move stage to data acquisition spot"
        # "CHANGE FISH FOR TETHER BACK\nTO TRUE VALUE HERE."
        n967 = event-data() -> ()  [unwired: 1 in, 5 out]
        n968 = local write "Cal/Data Acq. Spot"(FALSE ("Cal/Data Acq. Spot")) -> ()
        n969 = flat-sequence {
          tunnel: ["Cal @ (MHz)"] -> w5002
          tunnel: w5002 -> [w5012]
          tunnel: w5002 -> [w5033]
          frame #0 {
            n970 = property on="Trap Delta (MHz)" class="DigNum (strict)"("Val(Sgnl)"="Cal @ (MHz)") -> ()  [unwired: 2 in, 2 out]
            n971 = call <vilib>:"Beep.vi"() -> ()  [unwired: 3 in, 9 out]
          }
          frame #1 {
            n972 = Wait (ms)(milliseconds to wait=u32 100) -> ()  [unwired: 1 out]
          }
          frame #2 {
            n973 = property on="Save Calibration" class="Bool (strict)"("Val(Sgnl)"=TRUE ("Value (Signaling)")) -> ()  [unwired: 2 in, 2 out]
          }
          frame #3 {
            n974 = Wait (ms)(milliseconds to wait=u32 4000) -> ()  [unwired: 1 out]
          }
          frame #4 {
            n975 = while {
              stop <- w5009 stop-if-true
              n976 = local read "Saving..."() -> (w5010:bool)
              n977 = Wait (ms)(milliseconds to wait=u32 100) -> ()  [unwired: 1 out]
              n978 = Not(x=w5010) -> (.not. x?=w5009:bool)
            }
          }
          frame #5 {
            n979 = case shown="True" "W/ Offset 1" {
              tunnel: w5012 -> [_ w5014]
              frame False {
              }
              frame True {
                n980 = stacked-sequence {
                  tunnel: w5014 -> [_ _ _ _ _ _ _ w5031]
                  frame #0 {
                    n981 = Replace Array Subset(array=u32[] [0] ("Index Values"), new element="Offset 1 Set", index=0) -> (w5015:u32[])
                    n982 = property on="Saved AOD Raster Scan Parameter Sets" class="Arr (strict)"("Index Values"=w5015) -> ()  [unwired: 2 in, 2 out]
                    n983 = property on="Trap Delta (MHz)" class="DigNum (strict)"("Val(Sgnl)"="Offset 1 Start (MHz)") -> ()  [unwired: 2 in, 2 out]
                  }
                  frame #1 {
                    n984 = Wait (ms)(milliseconds to wait=u32 200) -> ()  [unwired: 1 out]
                  }
                  frame #2 {
                    n985 = property on="Load parameters" class="Bool (strict)"("Val(Sgnl)"=TRUE ("Value (Signaling)")) -> ()  [unwired: 2 in, 2 out]
                  }
                  frame #3 {
                    n986 = Wait (ms)(milliseconds to wait=u32 200) -> ()  [unwired: 1 out]
                  }
                  frame #4 {
                    n987 = property on="Trap Raster Scan" class="Bool (strict)"("Val(Sgnl)"=TRUE ("Value (Signaling)")) -> ()  [unwired: 2 in, 2 out]
                  }
                  frame #5 {
                    n988 = Wait (ms)(milliseconds to wait=u32 2000) -> ()  [unwired: 1 out]
                  }
                  frame #6 {
                    n989 = while {
                      stop <- w5028 stop-if-true
                      n990 = local read "Raster Scanning..."() -> (w5030:bool)
                      n991 = local read "Saving..."() -> (w5026:bool)
                      n992 = Wait (ms)(milliseconds to wait=u32 100) -> ()  [unwired: 1 out]
                      n993 = Not(x=w5026) -> (.not. x?=w5025:bool)
                      n994 = Not(x=w5030) -> (.not. x?=w5027:bool)
                      n995 = And(x=w5027, y=w5025) -> (x .and. y?=w5028:bool)
                    }
                  }
                  frame #7 {
                    n996 = property on="Trap Delta (MHz)" class="DigNum (strict)"("Val(Sgnl)"=w5031) -> ()  [unwired: 2 in, 2 out]
                  }
                }
              }
            }
          }
          frame #6 {
            n997 = local read "Save ave N"() -> (w5032:dbl)
            n998 = case shown="True" "W/ Offset 2" {
              tunnel: w5033 -> [_ w5039]
              tunnel: w5032 -> [_ w5038]
              frame False {
                n999 = Multiply(x="Cal read wait (s)", y=u32 1000 ("milliseconds to wait")) -> (x*y=w5036:u32)
                n1000 = Wait (ms)(milliseconds to wait=w5036) -> ()  [unwired: 1 out]
              }
              frame True {
                n1001 = stacked-sequence {
                  tunnel: w5039 -> [_ _ _ _ _ _ _ _ _ w5060 _ _]
                  tunnel: w5038 -> [_ _ _ _ _ _ _ _ _ w5058 _ _]
                  frame #0 {
                    n1002 = property on="Save ave N" class="DigNum (strict)"("Val(Sgnl)"=1.0 ("Value (Signaling)")) -> ()  [unwired: 2 in, 2 out]
                  }
                  frame #1 {
                    n1003 = Wait (ms)(milliseconds to wait=u32 500) -> ()  [unwired: 1 out]
                  }
                  frame #2 {
                    n1004 = property on="Trap Delta (MHz)" class="DigNum (strict)"("Val(Sgnl)"="Offset 2 Start (MHz)") -> ()  [unwired: 2 in, 2 out]
                    n1005 = Replace Array Subset(array=u32[] [0] ("Index Values"), new element="Offset 2 Set", index=0) -> (w5044:u32[])
                    n1006 = property on="Saved AOD Raster Scan Parameter Sets" class="Arr (strict)"("Index Values"=w5044) -> ()  [unwired: 2 in, 2 out]
                  }
                  frame #3 {
                    n1007 = Wait (ms)(milliseconds to wait=u32 500) -> ()  [unwired: 1 out]
                  }
                  frame #4 {
                    n1008 = property on="Load parameters" class="Bool (strict)"("Val(Sgnl)"=TRUE ("Value (Signaling)")) -> ()  [unwired: 2 in, 2 out]
                  }
                  frame #5 {
                    n1009 = Wait (ms)(milliseconds to wait=u32 500) -> ()  [unwired: 1 out]
                  }
                  frame #6 {
                    n1010 = property on="Trap Raster Scan" class="Bool (strict)"("Val(Sgnl)"=TRUE ("Value (Signaling)")) -> ()  [unwired: 2 in, 2 out]
                  }
                  frame #7 {
                    n1011 = Wait (ms)(milliseconds to wait=u32 2000) -> ()  [unwired: 1 out]
                  }
                  frame #8 {
                    n1012 = while {
                      stop <- w5053 stop-if-true
                      n1013 = local read "Raster Scanning..."() -> (w5056:bool)
                      n1014 = local read "Saving..."() -> (w5054:bool)
                      n1015 = Wait (ms)(milliseconds to wait=u32 100) -> ()  [unwired: 1 out]
                      n1016 = Not(x=w5054) -> (.not. x?=w5052:bool)
                      n1017 = Not(x=w5056) -> (.not. x?=w5055:bool)
                      n1018 = And(x=w5055, y=w5052) -> (x .and. y?=w5053:bool)
                    }
                  }
                  frame #9 {
                    n1019 = property on="Trap Delta (MHz)" class="DigNum (strict)"("Val(Sgnl)"=w5060) -> ()  [unwired: 2 in, 2 out]
                    n1020 = property on="Saved AOD Raster Scan Parameter Sets" class="Arr (strict)"("Index Values"=u32[] [0]) -> ()  [unwired: 2 in, 2 out]
                    n1021 = property on="Save ave N" class="DigNum (strict)"("Val(Sgnl)"=w5058) -> ()  [unwired: 2 in, 2 out]
                  }
                  frame #10 {
                    n1022 = Wait (ms)(milliseconds to wait=u32 500) -> ()  [unwired: 1 out]
                  }
                  frame #11 {
                    n1023 = property on="Load parameters" class="Bool (strict)"("Val(Sgnl)"=TRUE ("Value (Signaling)")) -> ()  [unwired: 2 in, 2 out]
                  }
                }
              }
            }
          }
          frame #7 {
            n1024 = property on="Read Cal" class="Bool (strict)"("Val(Sgnl)"=TRUE ("Value (Signaling)")) -> ()  [unwired: 2 in, 2 out]
          }
          frame #8 {
            n1025 = Wait (ms)(milliseconds to wait=u32 500) -> ()  [unwired: 1 out]
          }
          frame #9 {
            n1026 = property on="Fish for Tether" class="Bool (strict)"("Val(Sgnl)"=FALSE ("Value (Signaling)")) -> ()  [unwired: 2 in, 2 out]
          }
        }
      }
      event "Dump Beads": Value Change {
        # "SCRIPT TO REMOVE BOTH BEADS FROM THE TRAPS. TURNS ON LIGHT WHICH INDICATES THAT STAGE IS MOVING. THEN STOPS SAVING DATA. \nSETS Sample Channel Flow TO TRUE. STOPS INTERLACING GREEN FLUORESCENCE. TURNS OFF Tether INDICATOR BECAUSE WE ARE THROWING IT\nAWAY. SHUTS OFF TRAP POSITION FEEDBACK."
        n1027 = event-data() -> ()  [unwired: 1 in, 5 out]
        n1028 = flat-sequence {
          frame #0 {
            w5067 = FALSE ("Fl. Triggered...")
            w5068 = TRUE ("Stage Moving")
            n1029 = local read "Saving..."() -> (w5069:bool)
            n1030 = local write "Fl. Triggered..."(w5067) -> ()
            n1031 = local write "Stage Moving"(w5068) -> ()
            n1032 = local write "Tether"(w5067) -> ()
            n1033 = property on="Green Laser ON/Interlacing" class="Bool (strict)"("Val(Sgnl)"=w5067) -> ()  [unwired: 2 in, 2 out]
            n1034 = property on="Trap Pos. FB ON" class="Bool (strict)"("Val(Sgnl)"=w5067) -> ()  [unwired: 2 in, 2 out]
            n1035 = property on="Sample Channel Flow" class="Bool (strict)"("Val(Sgnl)"=w5068) -> ()  [unwired: 2 in, 2 out]
            n1036 = local write "Stop Saving"(w5069) -> ()
          }
          frame #1 {
            w5070 = FALSE ("Value (Signaling)")
            # "TURNS TRAPS OFF SO THAT\nBEADS REMAIN AT DUMP \nBEADS POSITION"
            n1037 = property on="Trap 1 (ON/OFF)" class="Bool (strict)"("Val(Sgnl)"=w5070) -> ()  [unwired: 2 in, 2 out]
            n1038 = property on="Trap 2 (ON/OFF)" class="Bool (strict)"("Val(Sgnl)"=w5070) -> ()  [unwired: 2 in, 2 out]
            n1039 = call <vilib>:"Beep.vi"() -> ()  [unwired: 3 in, 9 out]
          }
          frame #2 {
            n1040 = local read "Cal @ (MHz)"() -> (w5071:dbl)
            n1041 = property on="Trap Delta (MHz)" class="DigNum (strict)"("Val(Sgnl)"=w5071) -> ()  [unwired: 2 in, 2 out]
          }
        }
      }
      event "Dip for Protein": Value Change {
        n1042 = event-data() -> ()  [unwired: 1 in, 5 out]
        n1043 = flat-sequence {
          frame #0 {
            n1044 = case shown="True" "Move Trap Before?" {
              frame False {
              }
              frame True {
                n1045 = property on="Trap Delta (MHz)" class="DigNum (strict)"("Val(Sgnl)"="Dip Trap Delta 1 (MHz)") -> ()  [unwired: 2 in, 2 out]
              }
            }
          }
          frame #1 {
            n1046 = Multiply(x="Duration (s)", y=1000.0) -> (x*y=w5075:dbl)
            n1047 = Wait (ms)(milliseconds to wait=w5075) -> ()  [unwired: 1 out]
          }
          frame #2 {
            n1048 = case shown="True" "Move Trap After?" {
              frame False {
              }
              frame True {
                n1049 = property on="Trap Delta (MHz)" class="DigNum (strict)"("Val(Sgnl)"="Dip Trap Delta 2 (MHz)") -> ()  [unwired: 2 in, 2 out]
              }
            }
          }
          frame #3 {
            n1050 = case shown="True" "Green ON After?" {
              frame False {
              }
              frame True {
                n1051 = property on="Green Laser ON/Interlacing" class="Bool (strict)"("Val(Sgnl)"=TRUE ("Value (Signaling)")) -> ()  [unwired: 2 in, 2 out]
              }
            }
          }
          frame #4 {
            n1052 = Wait (ms)(milliseconds to wait=u32 500) -> ()  [unwired: 1 out]
          }
          frame #5 {
            n1053 = case shown="True" "Save Data After?" {
              frame False {
              }
              frame True {
                n1054 = property on="Start Saving" class="Bool (strict)"("Val(Sgnl)"=TRUE ("Value (Signaling)")) -> ()  [unwired: 2 in, 2 out]
              }
            }
          }
        }
      }
      event "Profile": Value Change {
        n1055 = event-data() -> ()  [unwired: 1 in, 5 out]
        n1056 = flat-sequence {
          frame #0 {
            w5085 = 0.0 ("element")
            n1057 = Build Array(w5085, "Y change (mm)", w5085) -> ()  [unwired: 1 out]
          }
          frame #1 {
            # "stop saving"
            n1058 = local write "Stop Saving"(TRUE ("Stop Saving")) -> ()
            n1059 = local write "Stage Moving"(FALSE ("Stage Moving")) -> ()
          }
        }
      }
      event "Got ADig bead": Value Change {
        n1060 = event-data() -> ()  [unwired: 1 in, 5 out]
        n1061 = property on="Move Cap. 1 (DNA Top)" class="Bool (strict)"("Val(Sgnl)"=TRUE ("Value (Signaling)")) -> ()  [unwired: 2 in, 2 out]
        n1062 = property on="Inject Bottom" class="Bool (strict)"("Val(Sgnl)"=FALSE ("Value (Signaling)")) -> ()  [unwired: 2 in, 2 out]
      }
      event "Got DNA bead": Value Change {
        n1063 = event-data() -> ()  [unwired: 1 in, 5 out]
        n1064 = property on="Cal/Data Acq. Spot" class="Bool (strict)"("Val(Sgnl)"=TRUE ("Value (Signaling)")) -> ()  [unwired: 2 in, 2 out]
        n1065 = property on="Inject Top" class="Bool (strict)"("Val(Sgnl)"=FALSE ("Value (Signaling)")) -> ()  [unwired: 2 in, 2 out]
      }
      event "Take Stepping Data": Value Change {
        n1066 = event-data() -> ()  [unwired: 1 in, 5 out]
        n1067 = local read "Save ave N"() -> (w5103:dbl)
        n1068 = flat-sequence {
          tunnel: w5103 -> [w5105]
          tunnel: [w5105] -> w5098
          tunnel: [w5107] -> w5099
          tunnel: w5098 -> [w5107]
          tunnel: [w5109] -> w5100
          tunnel: w5099 -> [w5109]
          tunnel: [w5112] -> w5101
          tunnel: w5100 -> [w5112]
          tunnel: [w5114] -> w5102
          tunnel: w5101 -> [w5114]
          tunnel: [w5116] -> w5096
          tunnel: w5102 -> [w5116]
          tunnel: w5096 -> [w5119]
          tunnel: [w5119] -> w5095
          tunnel: w5095 -> [w5120]
          tunnel: [w5120] -> w5097
          tunnel: w5097 -> [w5126]
          frame #0 {
            n1069 = property on="Save ave N" class="DigNum (strict)"("Val(Sgnl)"="Save ave factor") -> ()  [unwired: 2 in, 2 out]
          }
          frame #1 {
            n1070 = Wait (ms)(milliseconds to wait=u32 100) -> ()  [unwired: 1 out]
          }
          frame #2 {
            n1071 = local read "Offset 2 Start (MHz)"() -> (w5111:dbl)
            n1072 = property on="Saved AOD Raster Scan Parameter Sets" class="Arr (strict)"("Index Values"=u32[] [2]) -> ()  [unwired: 2 in, 2 out]
            n1073 = property on="Trap Delta (MHz)" class="DigNum (strict)"("Val(Sgnl)"=w5111) -> ()  [unwired: 2 in, 2 out]
          }
          frame #3 {
            n1074 = property on="Load parameters" class="Bool (strict)"("Val(Sgnl)"=TRUE ("Value (Signaling)")) -> ()  [unwired: 2 in, 2 out]
          }
          frame #4 {
            n1075 = Wait (ms)(milliseconds to wait=u32 100) -> ()  [unwired: 1 out]
          }
          frame #5 {
            n1076 = property on="Trap Raster Scan" class="Bool (strict)"("Val(Sgnl)"=TRUE ("Value (Signaling)")) -> ()  [unwired: 2 in, 2 out]
          }
          frame #6 {
            n1077 = Wait (ms)(milliseconds to wait=u32 1000) -> ()  [unwired: 1 out]
          }
          frame #7 {
            n1078 = while {
              stop <- w5123 stop-if-true
              n1079 = local read "Raster Scanning..."() -> (w5125:bool)
              n1080 = local read "Saving..."() -> (w5124:bool)
              n1081 = Not(x=w5124) -> (.not. x?=w5121:bool)
              n1082 = Not(x=w5125) -> (.not. x?=w5122:bool)
              n1083 = And(x=w5122, y=w5121) -> (x .and. y?=w5123:bool)
            }
          }
          frame #8 {
            n1084 = property on="Save ave N" class="DigNum (strict)"("Val(Sgnl)"=w5126) -> ()  [unwired: 2 in, 2 out]
          }
        }
      }
      event "Step Size (nm)": Value Change {
        n1085 = event-data() -> ()  [unwired: 1 in, 5 out]
        n1086 = flat-sequence {
          frame #0 {
            n1087 = property on="Saved AOD Raster Scan Parameter Sets" class="Arr (strict)"("Index Values"=u32[] [1]) -> ()  [unwired: 2 in, 2 out]
          }
          frame #1 {
            n1088 = Multiply(x="N Steps", y="Step Size (nm)") -> (x*y=w5128:dbl)
            n1089 = property on="Scan Speed AOD (nm/s) 2" class="DigNum (strict)"("Value"="Step Size (nm)") -> ()  [unwired: 2 in, 2 out]
            n1090 = property on="Step Size AOD (nm) 2" class="DigNum (strict)"("Value"="Step Size (nm)") -> ()  [unwired: 2 in, 2 out]
            n1091 = property on="Scan Range AOD (nm) 2" class="DigNum (strict)"("Value"=w5128) -> ()  [unwired: 2 in, 2 out]
          }
        }
      }
      event "Take Detection Laser\nImage": Value Change {
        n1092 = event-data() -> ()  [unwired: 1 in, 5 out]
        n1093 = flat-sequence {
          tunnel: [w5156] -> w5146
          tunnel: [w5155] -> w5139
          tunnel: [w5154] -> w5131
          tunnel: [w5159] -> w5147
          tunnel: w5146 -> [w5159]
          tunnel: [w5158] -> w5140
          tunnel: w5139 -> [w5158]
          tunnel: [w5157] -> w5132
          tunnel: w5131 -> [w5157]
          tunnel: [w5163] -> w5148
          tunnel: w5147 -> [w5163]
          tunnel: [w5162] -> w5141
          tunnel: w5140 -> [w5162]
          tunnel: [w5161] -> w5133
          tunnel: w5132 -> [w5161]
          tunnel: [w5169] -> w5149
          tunnel: w5148 -> [w5169]
          tunnel: [w5168] -> w5142
          tunnel: w5141 -> [w5168]
          tunnel: [w5167] -> w5134
          tunnel: w5133 -> [w5167]
          tunnel: [w5173] -> w5150
          tunnel: w5149 -> [w5173]
          tunnel: [w5172] -> w5143
          tunnel: w5142 -> [w5172]
          tunnel: [w5171] -> w5135
          tunnel: w5134 -> [w5171]
          tunnel: [w5177] -> w5151
          tunnel: w5150 -> [w5177]
          tunnel: [w5176] -> w5144
          tunnel: w5143 -> [w5176]
          tunnel: [w5175] -> w5136
          tunnel: w5135 -> [w5175]
          tunnel: [w5181] -> w5152
          tunnel: w5151 -> [w5181]
          tunnel: [w5180] -> w5145
          tunnel: w5144 -> [w5180]
          tunnel: [w5179] -> w5137
          tunnel: w5136 -> [w5179]
          tunnel: w5152 -> [w5187]
          tunnel: w5145 -> [w5186]